vi "NMR T2 CPMG Sequence - Small Magnet.vi"() -> ()   [LabVIEW 2020]
uses:
  <instrlib>/niFgen/niFgen.llb/niFgen Output Mode.ctl
  <instrlib>/niFgen/niFgen.llb/niFgen Waveform Type.ctl
  <instrlib>/niFgen/niFgen.llb/niFgen_ctl Trigger DigEdge - Edge Values (Ring).ctl
  <instrlib>/niFgen/niFgen.llb/niFgen_ctl Trigger Source Values (Ring).ctl
  <instrlib>/niFgen/niFgen.llb/niFgen Trigger Mode.ctl
  <instrlib>/niScope/Controls/niScope acquisition type.ctl
  <instrlib>/niScope/Controls/niScope trigger slope.ctl
  <instrlib>/niScope/Controls/niScope trigger source.ctl
  <vilib>/Analysis/2dsp.llb/Integral Method.ctl
  <vilib>/Analysis/8numeric.llb/1D Numeric Integration.vi
  <vilib>/Utility/file.llb/Read Delimited Spreadsheet (DBL).vi
  <instrlib>/niFgen/niFgen.llb/niFgen Create Waveform (DBL).vi
  <instrlib>/niScope/Configure/Trigger/niScope Configure Trigger Edge.vi
  <instrlib>/niFgen/niFgen.llb/niFgen Configure Digital Edge Start Trigger.vi
  <instrlib>/niScope/Acquire/Fetch/niScope Fetch Cluster.vi
  <vilib>/Waveform/WDTFileIO.llb/Export Waveform To Spreadsheet File.vi
  <vilib>/Analysis/NI_AALPro.lvlib
panel:
  out "Averaged T2 Decay":waveform(dbl)(graph)={"t0"=timestamp(0 s since 1904-01-01), "dt"=0.0012618296529968455, "Y"=array[3170 elements]} caption="Waveform Graph"
  out "Pulse Echos - Current Scan":T1(graph)={"relativeInitialX"=3.3333333333333337e-06, "xIncrement"=3.3333333333333333e-06, "wfm"=array[1260000 elements]} caption="Waveform Graph"
  in  "Write Output to File?":bool
  out "Scan Number":i32=1
  out "Signal Intensity (Integral)":dbl=0.6023718341213248 format="%0.4f"
  out "Extracted T2 Decay - Current Scan":waveform(dbl)(graph)={"t0"=timestamp(0 s since 1904-01-01), "dt"=0.0012618296529968455, "Y"=array[3170 elements]} caption="Waveform Graph"
  in  "Pulse Train File":path=path "D:/Pulse Train - 4s Duration, 3170 Pulses, 1.25ms Tau.txt"
  in  "Larmor Frequency":dbl=24028000.0 caption="Frequency" format="%.4p"
  in  "Number of Scans":i32=1
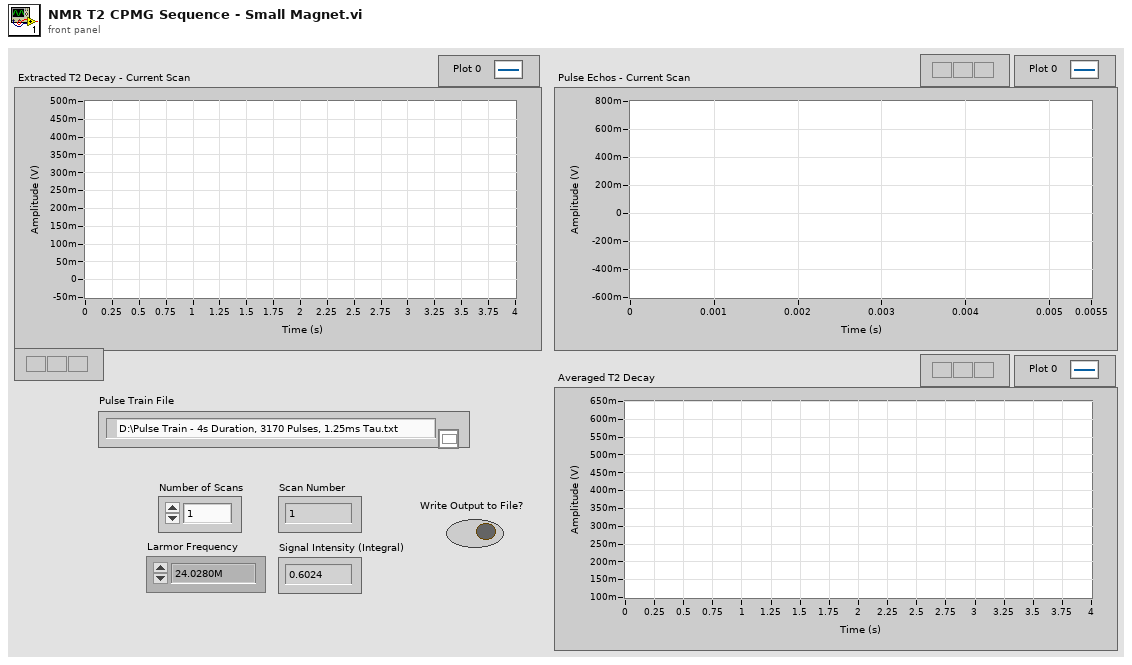
[diagram p1: front panel]
types:
  T1 = cluster{"relativeInitialX":dbl, "xIncrement":dbl, "wfm":dbl[]}
  T2 = typedef "niFgen Output Mode.ctl" = u32
  T3 = typedef "niScope trigger source.ctl" = string
  T4 = typedef "niFgen_ctl Trigger Source Values (Ring).ctl" = string
  T5 = typedef "NI_AALPro.lvlib/Integral Method.ctl" = i32
  T6 = typedef "niScope trigger slope.ctl" = i32
  T7 = typedef "niScope acquisition type.ctl" = i32
  T8 = typedef "niFgen Trigger Mode.ctl" = i32
  T9 = typedef "niFgen_ctl Trigger DigEdge - Edge Values (Ring).ctl" = i32
  T10 = typedef "niFgen Waveform Type.ctl" = i32
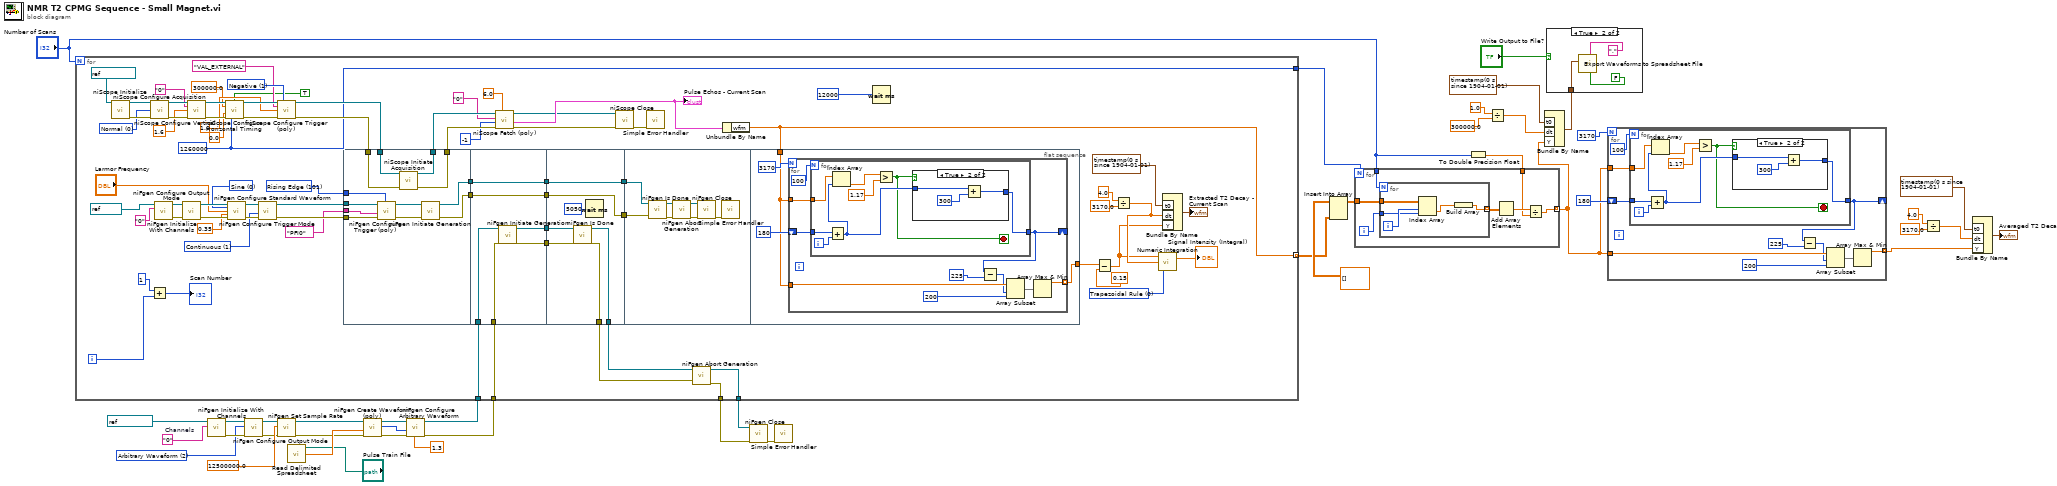
[diagram p0: block diagram]
diagram:
  w28 = "0"  # Channels
  w27 = T2 2 items=["Standard Function", "Frequency List", "Arbitrary Waveform", "Arbitrary Sequence", "Script"] ("output mode")
  n1 = call <instrlib>:"niFgen Initialize With Channels.vi"("Channel Name"=w28, "Resource Name"=refnum<k15> "PXI1Slot3" ("FGEN Resource Name 2")) -> ("error out"=w31:errorcluster, "Instrument Handle Out"=w32:refnum<k15>)  [unwired: 8 in]
  n2 = call <instrlib>:"niFgen Configure Output Mode.vi"("error in (no error)"=w31, "Output Mode (default: 0=Standard Function)"=w27, "Instrument Handle"=w32) -> ("error out"=w35:errorcluster, "Instrument Handle Out"=w34:refnum<k15>)  [unwired: 6 in]
  n3 = call <instrlib>:"niFgen Set Sample Rate.vi"("error in (no error)"=w35, "Sample Rate (Samp/s)"=12500000.0 ("Sample Rate"), "Instrument Handle"=w34) -> ("error out"=w38:errorcluster, "Instrument Handle Out"=w37:refnum<k15>)  [unwired: 7 in]
  n4 = call-poly <vilib>:"Read Delimited Spreadsheet.vi"("file path (dialog if empty)"="Pulse Train File") -> ("first row"=w39:dbl[])  [unwired: 9 in, 5 out]
  n5 = call-poly <instrlib>:"niFgen Create Waveform (poly).vi"("error in (no error)"=w38, "Waveform Data Array"=w39, "Instrument Handle"=w37) -> ("error out"=w41:errorcluster, "Waveform Handle"=w42:i32, "Instrument Handle Out"=w40:refnum<k15>)  [unwired: 6 in]
  n6 = call <instrlib>:"niFgen Configure Arbitrary Waveform.vi"("Gain"=1.3, "error in (no error)"=w41, "Waveform Handle"=w42, "Instrument Handle"=w40) -> ("error out"=w26:errorcluster, "Instrument Handle Out"=w25:refnum<k15>)  [unwired: 6 in]
  n7 = for {
    N: "Number of Scans" -> [_]
    tunnel: w26 -> [w99]
    tunnel: w25 -> [w98]
    tunnel: [w97] -> w23
    tunnel: [w96] -> w22
    tunnel: [w46] -> w19 mode=indexing
    tunnel: [w47] -> w10
    i -> [w54]
    w56 = T5 0 items=["Trapezoidal Rule", "Simpson's Rule", "Simpson's 3/8 Rule", "Bode Rule"] ("integration method")
    w47 = 1260000 ("min record length")
    w84 = T6 1 items=["Positive", "Negative"] ("trigger slope")
    w85 = T7 0 items=["Normal"=0, "Flex Res"=1, "DDC"=3] ("acquisition Type")
    w104 = T8 1 items=["Single", "Continuous", "Stepped", "Burst"] ("Trigger Mode (default: 1=continuous)")
    w108 = T9 101 items=["Rising Edge"=101, "Falling Edge"=102] ("Edge (Rising)")
    w109 = T10 0 items=["Sine", "Square", "Triangle", "Ramp Up", "Ramp Down", "DC", "Noise", "User"] ("Waveform")
    n8 = call <instrlib>:"niScope Initialize.vi"("resource name"=refnum<k15> "PXI1Slot6") -> ("instrument handle"=w86:refnum<k15>, "error out"=w87:errorcluster)  [unwired: 13 in]
    n9 = call <instrlib>:"niScope Configure Acquisition.vi"("instrument handle"=w86, "acquisition Type"=w85, "error in"=w87) -> ("instrument handle out"=w89:refnum<k15>, "error out"=w90:errorcluster)  [unwired: 11 in]
    n10 = Add(x=1, y=w54) -> (x+y=→"Scan Number":i32)
    n11 = call <instrlib>:"niFgen Initialize With Channels.vi"("Channel Name"="0", "Resource Name"=refnum<k15> "Dev1" ("Sine Wave Module")) -> ("error out"=w114:errorcluster, "Instrument Handle Out"=w117:refnum<k15>)  [unwired: 8 in]
    n12 = call <instrlib>:"niFgen Configure Output Mode.vi"("error in (no error)"=w114, "Instrument Handle"=w117) -> ("error out"=w113:errorcluster, "Instrument Handle Out"=w116:refnum<k15>)  [unwired: 7 in]
    n13 = call <instrlib>:"niScope Configure Vertical.vi"("instrument handle"=w89, "channels"="0", "vertical range"=1.6, "error in"=w90) -> ("instrument handle out"=w91:refnum<k15>, "error out"=w92:errorcluster)  [unwired: 10 in]
    n14 = call <instrlib>:"niScope Configure Horizontal Timing.vi"("instrument handle"=w91, "enforce realtime"=TRUE, "min sample rate"=300000.0, "reference position"=0.0, "error in"=w92, "min record length"=w47) -> ("instrument handle out"=w93:refnum<k15>, "error out"=w94:errorcluster)  [unwired: 8 in]
    n15 = call <instrlib>:"niFgen Configure Standard Waveform.vi"("Instrument Handle"=w116, "Waveform"=w109, "Frequency"="Larmor Frequency", "Amplitude"=0.35, "error in (no error)"=w113) -> ("Instrument Handle Out"=w115:refnum<k15>, "error out"=w112:errorcluster)  [unwired: 9 in]
    n16 = call <instrlib>:"niFgen Configure Trigger Mode.vi"("error in (no error)"=w112, "Trigger Mode (default: 1=continuous)"=w104, "Instrument Handle"=w115) -> ("error out"=w107:errorcluster, "Instrument Handle Out"=w105:refnum<k15>)  [unwired: 7 in]
    n17 = call-poly <instrlib>:"niScope Configure Trigger (poly).vi"("instrument handle"=w93, "trigger slope"=w84, "trigger source"=T3 "VAL_EXTERNAL", "trigger level"=1.0, "error in"=w94) -> ("instrument handle out"=w78:refnum<k15>, "error out"=w77:errorcluster)  [unwired: 9 in]
    n18 = flat-sequence {
      tunnel: w108 -> [w128]
      tunnel: w107 -> [w127]
      tunnel: T4 "PFI0" ("Source") -> [w126]
      tunnel: w105 -> [w125]
      tunnel: w78 -> [w123]
      tunnel: w77 -> [w122]
      tunnel: [w121] -> w76
      tunnel: [w120] -> w75
      tunnel: [w119] -> w65
      tunnel: [w118] -> w62
      tunnel: w99 -> [w135]
      tunnel: w98 -> [w134]
      tunnel: [w133] -> w69
      tunnel: [w132] -> w68
      tunnel: [w131] -> w66
      tunnel: w65 -> [w131]
      tunnel: [w130] -> w63
      tunnel: w62 -> [w130]
      tunnel: [w141] -> w102
      tunnel: [w140] -> w101
      tunnel: w69 -> [w139]
      tunnel: w68 -> [w138]
      tunnel: [w137] -> w67
      tunnel: w66 -> [w137]
      tunnel: [w136] -> w64
      tunnel: w63 -> [w136]
      tunnel: w67 -> [w144]
      tunnel: w64 -> [w143]
      tunnel: w46 -> [w150]
      tunnel: [w152] -> w44
      frame #0 {
        n19 = call-poly <instrlib>:"niFgen Configure Trigger (poly).vi"("Edge (Rising)"=w128, "error in (no error)"=w127, "Source"=w126, "Instrument Handle"=w125) -> ("error out"=w124:errorcluster, "Instrument Handle Out"=w129:refnum<k15>)  [unwired: 6 in]
        n20 = call <instrlib>:"niScope Initiate Acquisition.vi"("instrument handle"=w123, "error in"=w122) -> ("instrument handle out"=w121:refnum<k15>, "error out"=w120:errorcluster)  [unwired: 12 in]
        n21 = call <instrlib>:"niFgen Initiate Generation.vi"("error in (no error)"=w124, "Instrument Handle"=w129) -> ("error out"=w118:errorcluster, "Instrument Handle Out"=w119:refnum<k15>)  [unwired: 8 in]
      }
      frame #1 {
        n22 = call <instrlib>:"niFgen Initiate Generation.vi"("error in (no error)"=w135, "Instrument Handle"=w134) -> ("error out"=w132:errorcluster, "Instrument Handle Out"=w133:refnum<k15>)  [unwired: 8 in]
      }
      frame #2 {
        n23 = call <instrlib>:"niFgen Is Done.vi"("error in (no error)"=w138, "Instrument Handle"=w139) -> ("error out"=w141:errorcluster, "Instrument Handle Out"=w140:refnum<k15>)  [unwired: 7 in, 1 out]
        n24 = Wait (ms)(milliseconds to wait=u32 5050) -> ()  [unwired: 1 out]
      }
      frame #3 {
        n25 = call <instrlib>:"niFgen Is Done.vi"("error in (no error)"=w143, "Instrument Handle"=w144) -> ("error out"=w147:errorcluster, "Instrument Handle Out"=w146:refnum<k15>)  [unwired: 7 in, 1 out]
        n26 = call <instrlib>:"niFgen Abort Generation.vi"("error in (no error)"=w147, "Instrument Handle"=w146) -> ("error out"=w148:errorcluster, "Instrument Handle Out"=w149:refnum<k15>)  [unwired: 8 in]
        n27 = call <instrlib>:"niFgen Close.vi"("error in (no error)"=w148, "Instrument Handle"=w149) -> ("error out"=w145:errorcluster)  [unwired: 9 in]
        n28 = call <vilib>:"Simple Error Handler.vi"("error in (no error)"=w145) -> ()  [unwired: 4 in, 5 out]
      }
      frame #4 {
        n29 = for {
          N: 3170 -> [_]
          tunnel: [w162] -> w152 mode=indexing
          tunnel: w150 -> [w161]
          shift-right: [w156] -> _
          shift-left: 180 -> [w157]
          tunnel: w150 -> [w155]
          n30 = for {
            N: 100 -> [_]
            tunnel: w155 -> [w167]
            tunnel: w157 -> [w170]
            tunnel: [w165] -> w156
            i -> [w171]
            stop <- w164 stop-if-true
            n31 = Add(x=w170, y=w171) -> (x+y=w166:i32)
            n32 = Index Array(array=w167, index=w166) -> (element=w168:dbl)
            n33 = Greater?(x=w168, y=1.17) -> (0:w164:bool)
            n34 = case shown="True" w164 {
              tunnel: w166 -> [w172 w173]
              tunnel: [w172 w175] -> w165
              frame False {
              }
              frame True {
                n35 = Add(x=w173, y=300) -> (x+y=w175:i32)
              }
            }
          }
          n36 = Subtract(x=w156, y=225) -> (x-y=w158:i32)
          n37 = Array Subset(array=w161, index=w158, length=200 ("y")) -> (w163:dbl[])
          n38 = Array Max & Min(array=w163) -> (max value=w162:dbl)  [unwired: 3 out]
        }
      }
    }
    n39 = call-poly <instrlib>:"niScope Fetch (poly).vi"("timeout"=6.0, "error in"=w75, "numSamples"=-1, "channels"="0", "instrument handle"=w76) -> ("error out"=w48:errorcluster, "waveform"=w51:T1, "instrument handle out"=w49:refnum<k15>)  [unwired: 3 in, 1 out]
    "Pulse Echos - Current Scan" <- w51
    n40 = call <instrlib>:"niScope Close.vi"("instrument handle"=w49, "error in"=w48) -> ("error out"=w95:errorcluster)  [unwired: 13 in]
    n41 = call <vilib>:"Simple Error Handler.vi"("error in (no error)"=w95) -> ()  [unwired: 4 in, 5 out]
    n42 = call <instrlib>:"niFgen Abort Generation.vi"("error in (no error)"=w102, "Instrument Handle"=w101) -> ("error out"=w97:errorcluster, "Instrument Handle Out"=w96:refnum<k15>)  [unwired: 8 in]
    n43 = Unbundle By Name(w51) -> ("wfm"=w46:dbl[])
    n44 = Wait (ms)(milliseconds to wait=u32 12000 ("Delay Time (ms)")) -> ()  [unwired: 1 out]
    n45 = Subtract(x=w44, y=0.15) -> (x-y=w45:dbl[])
    n46 = Divide(x=4.0, y=3170.0) -> (x/y=w57:dbl)
    n47 = call-poly <vilib>:"Numeric Integration.vi"("integration method"=w56, "dt"=w57, "Input Array"=w45) -> ("result"=→"Signal Intensity (Integral)":dbl)  [unwired: 1 out]
    n48 = Bundle By Name("t0"=timestamp(0 s since 1904-01-01), "dt"=w57, "Y"=w45) -> (→"Extracted T2 Decay - Current Scan":waveform(dbl))  [unwired: 1 in]
  }
  n49 = call <instrlib>:"niFgen Close.vi"("error in (no error)"=w23, "Instrument Handle"=w22) -> ("error out"=w24:errorcluster)  [unwired: 9 in]
  n50 = call <vilib>:"Simple Error Handler.vi"("error in (no error)"=w24) -> ()  [unwired: 4 in, 5 out]
  n51 = Insert Into Array(array=dbl[][] [], new element=w19) -> (w21:dbl[][])  [unwired: 2 in]
  n52 = To Double Precision Float(number="Number of Scans") -> (double precision float=w18:dbl)
  n53 = for {
    N: w10 -> [_]
    tunnel: w21 -> [w182]
    tunnel: [w178] -> w2 mode=indexing
    tunnel: "Number of Scans" -> [w177]
    tunnel: w18 -> [w176]
    i -> [w181]
    n54 = for {
      N: w177 -> [_]
      tunnel: w182 -> [w187]
      tunnel: w181 -> [w185]
      tunnel: [w183] -> w180 mode=indexing
      i -> [w186]
      n55 = Index Array(array=w187, index (row)=w186, index (col)=w185) -> (element=w184:dbl)
      n56 = Build Array(w184) -> (w183:dbl[])
    }
    n57 = Add Array Elements(numeric array=w180) -> (sum=w179:dbl)
    n58 = Divide(x=w179, y=w176) -> (x/y=w178:dbl)
  }
  n59 = Divide(x=1.0, y=300000.0) -> (x/y=w13:dbl)
  n60 = Bundle By Name("t0"=timestamp(0 s since 1904-01-01), "dt"=w13, "Y"=w2) -> (w12:waveform(dbl))  [unwired: 1 in]
  n61 = case shown="True" "Write Output to File?" {
    tunnel: w12 -> [_ w188]
    frame False {
    }
    frame True {
      n62 = call-poly <vilib>:"Export Waveforms to Spreadsheet File.vi"("header? (write header:T)"=FALSE, "delimiter (Tab)"=",", "waveform"=w188) -> ()  [unwired: 7 in, 2 out]
    }
  }
  n63 = for {
    N: 3170 -> [_]
    tunnel: [w199] -> w1 mode=indexing
    tunnel: w2 -> [w198]
    shift-right: [w193] -> _
    shift-left: 180 -> [w194]
    tunnel: w2 -> [w192]
    n64 = for {
      N: 100 -> [_]
      tunnel: w192 -> [w204]
      tunnel: w194 -> [w207]
      tunnel: [w202] -> w193
      i -> [w208]
      stop <- w201 stop-if-true
      n65 = Add(x=w207, y=w208) -> (x+y=w203:i32)
      n66 = Index Array(array=w204, index=w203) -> (element=w205:dbl)
      n67 = Greater?(x=w205, y=1.17) -> (0:w201:bool)
      n68 = case shown="True" w201 {
        tunnel: w203 -> [w209 w210]
        tunnel: [w209 w212] -> w202
        frame False {
        }
        frame True {
          n69 = Add(x=w210, y=300) -> (x+y=w212:i32)
        }
      }
    }
    n70 = Subtract(x=w193, y=225) -> (x-y=w195:i32)
    n71 = Array Subset(array=w198, index=w195, length=200 ("y")) -> (w200:dbl[])
    n72 = Array Max & Min(array=w200) -> (max value=w199:dbl)  [unwired: 3 out]
  }
  n73 = Divide(x=4.0, y=3170.0) -> (x/y=w5:dbl)
  n74 = Bundle By Name("t0"=timestamp(0 s since 1904-01-01), "dt"=w5, "Y"=w1) -> (→"Averaged T2 Decay":waveform(dbl))  [unwired: 1 in]
